vi "Project-SmartHome.vi"() -> ()   [LabVIEW 2013] (continued)
      }
      event "play": Value Change {
        n589 = event-data() -> ()  [unwired: 1 in, 6 out]
        n590 = local read "flag 7"() -> (w1128:u16)
        n591 = local read "channel"() -> (w1129:dbl)
        n592 = Equal?(x=w1128, y=w1129) -> (x = y?=w1135:bool)
        n593 = case shown="False" w1135 {
          tunnel: w1134 -> [w1139 w1156]
          tunnel: w1133 -> [w1144 w1159]
          tunnel: w1132 -> [w1143 w1160]
          tunnel: [w1142 w1158] -> w1131
          tunnel: [w1141 w1157] -> w1130
          tunnel: w1128 -> [w1137 _]
          frame False {
            n594 = To Double Precision Float(number=w1137) -> (double precision float=w1136:dbl)
            n595 = local read "flag 7"() -> (→"channel":u16)
            n596 = local read "URL"() -> (w1154:string)
            n597 = property class="IWMPPlayer4"(reference=w1139, "URL"=w1154) -> (reference out=w1153:refnum<k7>)  [unwired: 1 in, 1 out]
            n598 = property class="IWMPPlayer4"(reference=w1153) -> ("controls"=w1152:refnum<k7>)  [unwired: 1 in, 2 out]
            n599 = invoke class="IWMPControls" method="play"(reference=w1152) -> (reference out=w1151:refnum<k7>)  [unwired: 2 in, 2 out]
            n600 = Type Cast(x=8.0) -> (*(type *) &x=w1145:string)  [unwired: 1 in]
            n601 = TCP Write(connection ID=w1144, data in=w1145, error in (no error)=w1143) -> (connection ID out=w1147:refnum<k5>, error out=w1148:errorcluster)  [unwired: 1 in, 1 out]
            n602 = Close Reference(reference=w1151) -> ()  [unwired: 1 in, 1 out]
            n603 = Bundle(w1136, 1.0) -> (w1149:cluster{dbl, dbl})  [unwired: 1 in]
            n604 = Type Cast(x=w1149) -> (*(type *) &x=w1150:string)  [unwired: 1 in]
            n605 = TCP Write(connection ID=w1147, data in=w1150, error in (no error)=w1148) -> (connection ID out=w1142:refnum<k5>, error out=w1141:errorcluster)  [unwired: 1 in, 1 out]
          }
          frame True {
            n606 = property class="IWMPPlayer4"(reference=w1156) -> ("controls"=w1167:refnum<k7>)  [unwired: 1 in, 2 out]
            n607 = invoke class="IWMPControls" method="play"(reference=w1167) -> (reference out=w1168:refnum<k7>)  [unwired: 2 in, 2 out]
            n608 = Type Cast(x=7.0) -> (*(type *) &x=w1161:string)  [unwired: 1 in]
            n609 = TCP Write(connection ID=w1159, data in=w1161, error in (no error)=w1160) -> (connection ID out=w1163:refnum<k5>, error out=w1164:errorcluster)  [unwired: 1 in, 1 out]
            n610 = Bundle(2.0) -> (w1165:cluster{dbl})  [unwired: 1 in]
            n611 = Type Cast(x=w1165) -> (*(type *) &x=w1166:string)  [unwired: 1 in]
            n612 = Close Reference(reference=w1168) -> ()  [unwired: 1 in, 1 out]
            n613 = TCP Write(connection ID=w1163, data in=w1166, error in (no error)=w1164) -> (connection ID out=w1158:refnum<k5>, error out=w1157:errorcluster)  [unwired: 1 in, 1 out]
          }
        }
      }
      event "flag 7": Value Change {
        n614 = event-data() -> ()  [unwired: 1 in, 6 out]
        n615 = case shown="2" "flag 7" {
          frame 0, Default {
            "URL" <- "C:\\Users\\kiat\\Downloads\\asd.mp4" ("URL")
          }
          frame 1 {
            n616 = local write "URL"("C:\\Users\\kiat\\Downloads\\videoplayback.mp4" ("URL")) -> ()
          }
          frame 2 {
            n617 = local write "URL"("C:\\Users\\kiat\\Downloads\\wiggle.mp4" ("URL")) -> ()
          }
        }
      }
      event "backward": Value Change {
        n618 = event-data() -> ()  [unwired: 1 in, 6 out]
        n619 = Automation Open(Automation Refnum=w1185) -> (Automation Refnum=w1186:refnum<k7>)  [unwired: 3 in, 1 out]
        n620 = property class="IWMPPlayer4"(reference=w1186) -> ("controls"=w1187:refnum<k7>)  [unwired: 1 in, 2 out]
        n621 = invoke class="IWMPControls" method="fastReverse"(reference=w1187) -> (reference out=w1184:refnum<k7>)  [unwired: 2 in, 2 out]
        n622 = Type Cast(x=7.0) -> (*(type *) &x=w1178:string)  [unwired: 1 in]
        n623 = TCP Write(connection ID=w1176, data in=w1178, error in (no error)=w1175) -> (connection ID out=w1180:refnum<k5>, error out=w1181:errorcluster)  [unwired: 1 in, 1 out]
        n624 = Close Reference(reference=w1184) -> ()  [unwired: 1 in, 1 out]
        n625 = Bundle(5.0) -> (w1182:cluster{dbl})  [unwired: 1 in]
        n626 = Type Cast(x=w1182) -> (*(type *) &x=w1183:string)  [unwired: 1 in]
        n627 = TCP Write(connection ID=w1180, data in=w1183, error in (no error)=w1181) -> (connection ID out=w1174:refnum<k5>, error out=w1173:errorcluster)  [unwired: 1 in, 1 out]
      }
      event "foward": Value Change {
        n628 = event-data() -> ()  [unwired: 1 in, 6 out]
        n629 = Type Cast(x=7.0) -> (*(type *) &x=w1193:string)  [unwired: 1 in]
        n630 = TCP Write(connection ID=w1191, data in=w1193, error in (no error)=w1190) -> (connection ID out=w1195:refnum<k5>, error out=w1196:errorcluster)  [unwired: 1 in, 1 out]
        n631 = Bundle(6.0) -> (w1197:cluster{dbl})  [unwired: 1 in]
        n632 = Type Cast(x=w1197) -> (*(type *) &x=w1198:string)  [unwired: 1 in]
        n633 = TCP Write(connection ID=w1195, data in=w1198, error in (no error)=w1196) -> (connection ID out=w1189:refnum<k5>, error out=w1188:errorcluster)  [unwired: 1 in, 1 out]
        n634 = Automation Open(Automation Refnum=w1200) -> (Automation Refnum=w1201:refnum<k7>)  [unwired: 3 in, 1 out]
        n635 = property class="IWMPPlayer4"(reference=w1201) -> ("controls"=w1202:refnum<k7>)  [unwired: 1 in, 2 out]
        n636 = invoke class="IWMPControls" method="fastForward"(reference=w1202) -> (reference out=w1199:refnum<k7>)  [unwired: 2 in, 2 out]
        n637 = Close Reference(reference=w1199) -> ()  [unwired: 1 in, 1 out]
      }
      event "pause": Value Change {
        n638 = event-data() -> ()  [unwired: 1 in, 6 out]
        n639 = Automation Open(Automation Refnum=w1215) -> (Automation Refnum=w1214:refnum<k7>)  [unwired: 3 in, 1 out]
        n640 = property class="IWMPPlayer4"(reference=w1214) -> ("controls"=w1217:refnum<k7>)  [unwired: 1 in, 2 out]
        n641 = invoke class="IWMPControls" method="pause"(reference=w1217) -> (reference out=w1216:refnum<k7>)  [unwired: 2 in, 2 out]
        n642 = Type Cast(x=7.0) -> (*(type *) &x=w1208:string)  [unwired: 1 in]
        n643 = TCP Write(connection ID=w1203, data in=w1208, error in (no error)=w1204) -> (connection ID out=w1210:refnum<k5>, error out=w1211:errorcluster)  [unwired: 1 in, 1 out]
        n644 = Close Reference(reference=w1216) -> ()  [unwired: 1 in, 1 out]
        n645 = Bundle(3.0) -> (w1212:cluster{dbl})  [unwired: 1 in]
        n646 = Type Cast(x=w1212) -> (*(type *) &x=w1213:string)  [unwired: 1 in]
        n647 = TCP Write(connection ID=w1210, data in=w1213, error in (no error)=w1211) -> (connection ID out=w1206:refnum<k5>, error out=w1205:errorcluster)  [unwired: 1 in, 1 out]
      }
      event "add": Value Change {
        n648 = event-data() -> ()  [unwired: 1 in, 6 out]
        n649 = Read from Text File(file (use dialog)=w1219) -> (refnum out=w1220:refnum<file>, text=w1218:string)  [unwired: 3 in, 2 out]
        n650 = while {
          tunnel: w1218 -> [w1224]
          border: w1218 -> [_]
          stop <- w1222 stop-if-true
          n651 = feedback #1() -> (w1230:string)
          n652 = xnode "Match Regular Expression"("input string"=w1230, "regular expression"="\n") -> ("before match"=w1227:string, "after match"=w1231:string)  [unwired: 4 in, 3 out]
          n653 = feedback-in #1(w1231) -> ()
          n654 = Empty String/Path?(string/path=w1231) -> (empty?=w1221:bool)
          n655 = xnode "Match Regular Expression"("input string"=w1227, "regular expression"="-") -> ("before match"=w1228:string)  [unwired: 4 in, 4 out]
          n656 = local read "String"() -> (w1223:string)
          n657 = Equal?(x=w1223, y=w1228) -> (x = y?=w1225:bool)
          n658 = case shown="False" w1225 {
            tunnel: w1224 -> [w1233 _]
            tunnel: [w1232 w1261] -> w1222
            tunnel: w1221 -> [w1232 _]
            frame False {
              n659 = case shown="True" w1232 {
                tunnel: w1233 -> [_ w1238]
                frame False {
                }
                frame True {
                  n660 = case shown="1" "flag 8" {
                    tunnel: [w1259 w1260] -> w1242
                    tunnel: [w1259 w1260] -> w1246
                    frame 0, Default {
                      w1259 = "Admin"
                    }
                    frame 1 {
                      w1260 = "User"
                    }
                  }
                  n661 = Concatenate Strings("String", "-" ("string"), "String", ":" ("string"), w1242) -> (w1250:string)
                  n662 = local read "Numeric"() -> (w1249:dbl)
                  n663 = Open/Create/Replace File(file path (use dialog)=path "C:/Users/kiat/Desktop/password.txt" ("file (use dialog)")) -> (refnum out=w1236:refnum<file>)  [unwired: 5 in, 2 out]
                  n664 = local read "Table Control"() -> (w1247:string[][])
                  n665 = Build Array("String", "String", w1246) -> (w1243:string[])
                  n666 = case shown="0, Default" w1249 {
                    tunnel: [w1252 w1258] -> w1235
                    tunnel: w1238 -> [w1254 w1257]
                    tunnel: w1250 -> [w1253 w1255]
                    frame 0, Default {
                      n667 = Concatenate Strings(w1254, w1253) -> (w1252:string)
                      n668 = local write "Numeric"(0.0) -> ()
                    }
                    frame 1 {
                      n669 = Concatenate Strings(w1257, "\n", w1255) -> (w1258:string)
                    }
                  }
                  n670 = Write to Text File(file (use dialog)=w1236, text=w1235) -> (refnum out=w1237:refnum<file>)  [unwired: 2 in, 2 out]
                  n671 = Insert Into Array(array=w1247, new element=w1243) -> (w1248:string[][])  [unwired: 2 in]
                  n672 = local write "Table Control"(w1248) -> ()
                  n673 = Close File(refnum=w1237) -> ()  [unwired: 1 in, 2 out]
                }
              }
            }
            frame True {
              n674 = call "Display Message to User2"("Message"="Please choose another name") -> ("OK"=w1261:bool)  [unwired: 9 in, 1 out]
            }
          }
        }
        n675 = Close File(refnum=w1220) -> ()  [unwired: 1 in, 2 out]
      }
      event "edit": Value Change {
        n676 = event-data() -> ()  [unwired: 1 in, 6 out]
        n677 = property on="Table Control" class="Tbl (strict)"() -> ("Value"=w1486:string[][])  [unwired: 2 in, 2 out]
        n678 = local read "String"() -> (w1494:string)
        n679 = Read from Text File(file (use dialog)=w1493) -> (refnum out=w1507:refnum<file>, text=w1489:string, error out=w1513:errorcluster)  [unwired: 3 in, 1 out]
        n680 = Decimal String To Number(string=w1494) -> (number=w1487:i32)  [unwired: 2 in, 1 out]
        n681 = local read "Table Control"() -> (w1500:string[][])
        n682 = Array Size(array=w1486) -> (size(s)=w1496:i32[])
        n683 = local read "String"() -> (w1497:string)
        n684 = Add(x=1, y=w1487) -> (x+y=w1488:i32)
        n685 = Close File(refnum=w1507, error in=w1513) -> (path=w1504:path, error out=w1503:errorcluster)
        n686 = Index Array(array=w1496) -> (element=w1495:i32)  [unwired: 1 in]
        n687 = Decimal String To Number(string=w1497) -> (number=w1491:i32)  [unwired: 2 in, 1 out]
        n688 = Greater Or Equal?(x=w1488, y=w1495) -> (x >= y?=w1485:bool)
        n689 = case shown="True" w1485 {
          frame False {
          }
          frame True {
            n690 = local write "Table Control"(string[][] [] ("Table Control")) -> ()
            n691 = Read from Text File(file (use dialog)=path "C:/Users/kiat/Desktop/password.txt") -> (text=w1516:string)  [unwired: 3 in, 3 out]
            n692 = while {
              border: w1516 -> [_]
              stop <- w1526 stop-if-true
              n693 = feedback #2() -> (w1530:string)
              n694 = xnode "Match Regular Expression"("input string"=w1530, "regular expression"="\n") -> ("before match"=w1529:string, "after match"=w1528:string)  [unwired: 4 in, 3 out]
              n695 = feedback-in #2(w1528) -> ()
              n696 = xnode "Match Regular Expression"("input string"=w1529, "regular expression"="-") -> ("before match"=w1525:string, "after match"=w1524:string)  [unwired: 4 in, 3 out]
              n697 = Equal?(x=w1528, y="") -> (x = y?=w1526:bool)
              n698 = xnode "Match Regular Expression"("input string"=w1524, "regular expression"=":") -> ("before match"=w1521:string, "after match"=w1522:string)  [unwired: 4 in, 3 out]
              n699 = local read "Table Control"() -> (w1518:string[][])
              n700 = Build Array(w1525, w1521, w1522) -> (w1520:string[])
              n701 = Insert Into Array(array=w1518, new element=w1520) -> (w1519:string[][])  [unwired: 2 in]
              n702 = local write "Table Control"(w1519) -> ()
            }
          }
        }
        n703 = Index Array(array=w1500, index (row)=w1491, index (col)=0 ("index")) -> (element=w1502:string)
        n704 = local read "String"() -> (w1498:string)
        n705 = local read "Table Control"() -> (w1499:string[][])
        n706 = Open/Create/Replace File(file path (use dialog)=w1504, error in=w1503, operation (0:open)=T2."replace") -> (refnum out=w1511:refnum<file>, error out=w1510:errorcluster)  [unwired: 3 in, 1 out]
        n707 = Decimal String To Number(string=w1498) -> (number=w1492:i32)  [unwired: 2 in, 1 out]
        n708 = Index Array(array=w1499, index (row)=w1492, index (col)=1 ("index")) -> (element=w1508:string)
        n709 = while {
          tunnel: w1502 -> [w1889]
          tunnel: w1508 -> [w1888]
          border: "" -> [_]
          tunnel: [w1884] -> w1506
          border: w1489 -> [_]
          stop <- w1893 stop-if-true
          n710 = feedback #3() -> (w1891:string)
          n711 = xnode "Match Regular Expression"("input string"=w1891, "regular expression"="\n") -> ("before match"=w1887:string, "after match"=w1892:string)  [unwired: 4 in, 3 out]
          n712 = feedback-in #3(w1892) -> ()
          n713 = Empty String/Path?(string/path=w1892) -> (empty?=w1893:bool)
          n714 = xnode "Match Regular Expression"("input string"=w1887, "regular expression"="-") -> ("before match"=w1881:string, "after match"=w1883:string)  [unwired: 4 in, 3 out]
          n715 = xnode "Match Regular Expression"("input string"=w1883, "regular expression"=":") -> ("before match"=w1880:string)  [unwired: 4 in, 4 out]
          n716 = local read "flag 8"() -> (w1876:u16)
          n717 = case shown="1" w1876 {
            tunnel: ["Admin" "User"] -> w1875
            frame 0, Default {
            }
            frame 1 {
            }
          }
          n718 = Equal?(x=w1889, y=w1881) -> (x = y?=w1879:bool)
          n719 = Equal?(x=w1888, y=w1880) -> (x = y?=w1878:bool)
          n720 = And(x=w1879, y=w1878) -> (x .and. y?=w1877:bool)
          n721 = case shown="True" w1877 {
            tunnel: w1887 -> [w2009 w2018]
            tunnel: [w2008 w2017] -> w1886
            tunnel: w1875 -> [_ w2011]
            frame False {
              n722 = Concatenate Strings(w2009, "\n") -> (w2008:string)
            }
            frame True {
              n723 = local read "String"() -> (w2016:string)
              n724 = local read "String"() -> (w2014:string)
              n725 = Concatenate Strings(w2016, "-" ("string"), w2014, ":" ("string"), w2011) -> (w2012:string)
              n726 = Search and Replace String(input string=w2018, search string=w2018, replace string=w2012) -> (result string=w2017:string)  [unwired: 5 in, 3 out]
            }
          }
          n727 = feedback #4() -> (w1885:string)
          n728 = Concatenate Strings(w1885, w1886) -> (w1884:string)
          n729 = feedback-in #4(w1884) -> ()
        }
        n730 = Write to Text File(file (use dialog)=w1511, text=w1506, error in=w1510) -> (refnum out=w1505:refnum<file>)  [unwired: 1 in, 2 out]
        n731 = Close File(refnum=w1505) -> ()  [unwired: 1 in, 2 out]
      }
      event "delete": Value Change {
        n732 = event-data() -> ()  [unwired: 1 in, 6 out]
        n733 = property on="Table Control" class="Tbl (strict)"() -> ("Value"=w2245:string[][])  [unwired: 2 in, 2 out]
        n734 = Read from Text File(file (use dialog)=w2249) -> (refnum out=w2256:refnum<file>, text=w2261:string, error out=w2265:errorcluster)  [unwired: 3 in, 1 out]
        n735 = local read "String"() -> (w2251:string)
        n736 = Decimal String To Number(string=w2251) -> (number=w2250:i32)  [unwired: 2 in, 1 out]
        n737 = Array Size(array=w2245) -> (size(s)=w2254:i32[])
        n738 = local read "String"() -> (w2266:string)
        n739 = Index Array(array=w2254) -> (element=w2253:i32)  [unwired: 1 in]
        n740 = local read "Table Control"() -> (w2247:string[][])
        n741 = Close File(refnum=w2256, error in=w2265) -> (path=w2244:path, error out=w2243:errorcluster)
        n742 = Greater Or Equal?(x=w2250, y=w2253) -> (x >= y?=w2252:bool)
        n743 = Decimal String To Number(string=w2266) -> (number=w2268:i32)  [unwired: 2 in, 1 out]
        n744 = Index Array(array=w2247, index (row)=w2268, index (col)=0 ("index")) -> (element=w2242:string)
        n745 = case shown="False" w2252 {
          tunnel: w2250 -> [w2271 _]
          tunnel: w2245 -> [w2270 _]
          frame False {
            n746 = Delete From Array(array=w2270, length=1, index (row)=w2271) -> (array with subset deleted=w2269:string[][])  [unwired: 1 in, 1 out]
            n747 = property on="Table Control" class="Tbl (strict)"("Value"=w2269) -> ()  [unwired: 2 in, 2 out]
          }
          frame True {
          }
        }
        n748 = local read "String"() -> (w2260:string)
        n749 = local read "Table Control"() -> (w2246:string[][])
        n750 = Open/Create/Replace File(file path (use dialog)=w2244, error in=w2243, operation (0:open)=T2."replace") -> (refnum out=w2263:refnum<file>, error out=w2262:errorcluster)  [unwired: 3 in, 1 out]
        n751 = Decimal String To Number(string=w2260) -> (number=w2258:i32)  [unwired: 2 in, 1 out]
        n752 = Index Array(array=w2246, index (row)=w2258, index (col)=1 ("index")) -> (element=w2257:string)
        n753 = while {
          tunnel: w2261 -> [w2289]
          tunnel: w2242 -> [w2286]
          tunnel: w2257 -> [w2285]
          border: "" -> [_]
          tunnel: [w2278] -> w2255
          stop <- w2292 stop-if-true
          n754 = Wait Until Next ms Multiple(millisecond multiple=u32 2000) -> ()  [unwired: 1 out]
          n755 = feedback #5(w2289) -> (w2290:string)
          n756 = xnode "Match Regular Expression"("input string"=w2290, "regular expression"="\n") -> ("before match"=w2281:string, "after match"=w2291:string)  [unwired: 4 in, 3 out]
          n757 = feedback-in #5(w2291) -> ()
          n758 = Empty String/Path?(string/path=w2291) -> (empty?=w2292:bool)
          n759 = xnode "Match Regular Expression"("input string"=w2281, "regular expression"="-") -> ("before match"=w2287:string, "after match"=w2276:string)  [unwired: 4 in, 3 out]
          n760 = xnode "Match Regular Expression"("input string"=w2276, "regular expression"=":") -> ("before match"=w2274:string)  [unwired: 4 in, 4 out]
          n761 = Equal?(x=w2286, y=w2287) -> (x = y?=w2283:bool)
          n762 = Equal?(x=w2285, y=w2274) -> (x = y?=w2284:bool)
          n763 = And(x=w2283, y=w2284) -> (x .and. y?=w2282:bool)
          n764 = case shown="False" w2282 {
            tunnel: w2281 -> [w2406 w2410]
            tunnel: [w2405 w2408] -> w2280
            frame False {
              n765 = Concatenate Strings(w2406, "\n") -> (w2405:string)
            }
            frame True {
              n766 = Search and Replace String(input string=w2410, search string=w2410, replace string="" ("replace string (\"\")")) -> (result string=w2408:string)  [unwired: 5 in, 3 out]
            }
          }
          n767 = local write "Numeric"(0.0 ("Numeric")) -> ()
          n768 = feedback #6() -> (w2279:string)
          n769 = Concatenate Strings(w2279, w2280) -> (w2278:string)
          n770 = feedback-in #6(w2278) -> ()
        }
        n771 = Write to Text File(file (use dialog)=w2263, text=w2255, error in=w2262) -> (refnum out=w2248:refnum<file>)  [unwired: 1 in, 2 out]
        n772 = Close File(refnum=w2248) -> ()  [unwired: 1 in, 2 out]
      }
      event Value Change {
        n773 = event-data() -> ()  [unwired: 1 in, 6 out]
        n774 = property class="IWMPPlayer4"(reference=w2646) -> ("settings"=w2647:refnum<k7>)  [unwired: 1 in, 2 out]
        n775 = Type Cast(x=8.0) -> (*(type *) &x=w2639:string)  [unwired: 1 in]
        n776 = TCP Write(connection ID=w2638, data in=w2639, error in (no error)=w2637) -> (connection ID out=w2641:refnum<k5>, error out=w2642:errorcluster)  [unwired: 1 in, 1 out]
        n777 = Bundle("?", 2.0) -> (w2643:cluster{dbl, dbl})  [unwired: 1 in]
        n778 = Type Cast(x=w2643) -> (*(type *) &x=w2644:string)  [unwired: 1 in]
        n779 = TCP Write(connection ID=w2641, data in=w2644, error in (no error)=w2642) -> (connection ID out=w2636:refnum<k5>, error out=w2635:errorcluster)  [unwired: 1 in, 1 out]
        n780 = property class="IWMPSettings"(reference=w2647, "volume"="?") -> (reference out=w2645:refnum<k7>)  [unwired: 1 in, 1 out]
        n781 = Close Reference(reference=w2645) -> ()  [unwired: 1 in, 1 out]
      }
      event Value Change {
        n782 = event-data() -> ()  [unwired: 1 in, 6 out]
        n783 = property on="Tab Control" class="TabCtl (strict)"("Visible"=FALSE) -> ()  [unwired: 2 in, 2 out]
        n784 = property on="Tab Control 2" class="TabCtl (strict)"("Visible"=FALSE) -> ()  [unwired: 2 in, 2 out]
        n785 = property on="Tab Control 3" class="TabCtl (strict)"("Visible"=FALSE) -> ()  [unwired: 2 in, 2 out]
        n786 = property on="Tab Control 4" class="TabCtl (strict)"("Visible"=FALSE) -> ()  [unwired: 2 in, 2 out]
        n787 = property on="Tab Control 5" class="TabCtl (strict)"("Visible"=FALSE) -> ()  [unwired: 2 in, 2 out]
        n788 = property on="Tab Control 11" class="TabCtl (strict)"("Visible"=FALSE) -> ()  [unwired: 2 in, 2 out]
        n789 = property on="Tab Control 6" class="TabCtl (strict)"("Visible"=FALSE) -> ()  [unwired: 2 in, 2 out]
        n790 = property on="Tab Control 10" class="TabCtl (strict)"("Visible"=FALSE) -> ()  [unwired: 2 in, 2 out]
        n791 = property on="Tab Control 13" class="TabCtl (strict)"("Visible"=FALSE) -> ()  [unwired: 2 in, 2 out]
        n792 = property on="Tab Control 7" class="TabCtl (strict)"("Visible"=FALSE) -> ()  [unwired: 2 in, 2 out]
        n793 = property on="Tab Control 12" class="TabCtl (strict)"("Visible"=FALSE) -> ()  [unwired: 2 in, 2 out]
        n794 = property on="Tab Control 8" class="TabCtl (strict)"("Visible"=FALSE) -> ()  [unwired: 2 in, 2 out]
        n795 = property on="Tab Control 9" class="TabCtl (strict)"("Visible"=FALSE) -> ()  [unwired: 2 in, 2 out]
        n796 = property on="Tab Control 25" class="TabCtl (strict)"("Visible"=TRUE) -> ()  [unwired: 2 in, 2 out]
        n797 = property on="Tab Control 15" class="TabCtl (strict)"("Visible"=FALSE) -> ()  [unwired: 2 in, 2 out]
        n798 = property on="Tab Control 24" class="TabCtl (strict)"("Visible"=FALSE) -> ()  [unwired: 2 in, 2 out]
        n799 = property on="Tab Control 21" class="TabCtl (strict)"("Visible"=FALSE) -> ()  [unwired: 2 in, 2 out]
        n800 = property on="Tab Control 16" class="TabCtl (strict)"("Visible"=FALSE) -> ()  [unwired: 2 in, 2 out]
        n801 = property on="Tab Control 17" class="TabCtl (strict)"("Visible"=FALSE) -> ()  [unwired: 2 in, 2 out]
        n802 = property on="Tab Control 22" class="TabCtl (strict)"("Visible"=FALSE) -> ()  [unwired: 2 in, 2 out]
        n803 = property on="Tab Control 23" class="TabCtl (strict)"("Visible"=FALSE) -> ()  [unwired: 2 in, 2 out]
        n804 = property on="Tab Control 18" class="TabCtl (strict)"("Visible"=FALSE) -> ()  [unwired: 2 in, 2 out]
        n805 = property on="Tab Control 19" class="TabCtl (strict)"("Visible"=FALSE) -> ()  [unwired: 2 in, 2 out]
        n806 = property on="Tab Control 14" class="TabCtl (strict)"("Visible"=FALSE) -> ()  [unwired: 2 in, 2 out]
      }
      event "stop": Value Change {
        n807 = event-data() -> ()  [unwired: 1 in, 6 out]
        n808 = Type Cast(x=7.0) -> (*(type *) &x=w2677:string)  [unwired: 1 in]
        n809 = TCP Write(connection ID=w2675, data in=w2677, error in (no error)=w2674) -> (connection ID out=w2679:refnum<k5>, error out=w2680:errorcluster)  [unwired: 1 in, 1 out]
        n810 = Automation Open(Automation Refnum=w2684) -> (Automation Refnum=w2685:refnum<k7>)  [unwired: 3 in, 1 out]
        n811 = property class="IWMPPlayer4"(reference=w2685) -> ("controls"=w2686:refnum<k7>)  [unwired: 1 in, 2 out]
        n812 = invoke class="IWMPControls" method="stop"(reference=w2686) -> (reference out=w2683:refnum<k7>)  [unwired: 2 in, 2 out]
        n813 = Bundle(4.0) -> (w2681:cluster{dbl})  [unwired: 1 in]
        n814 = Type Cast(x=w2681) -> (*(type *) &x=w2682:string)  [unwired: 1 in]
        n815 = Close Reference(reference=w2683) -> ()  [unwired: 1 in, 1 out]
        n816 = TCP Write(connection ID=w2679, data in=w2682, error in (no error)=w2680) -> (connection ID out=w2673:refnum<k5>, error out=w2672:errorcluster)  [unwired: 1 in, 1 out]
      }
      event Value Change {
        # "Air conditional - Master room (set temperature)"
        n817 = event-data() -> ()  [unwired: 1 in, 6 out]
        n818 = Decimal String To Number(string="String") -> (number=w2693:i32)  [unwired: 2 in, 1 out]
        n819 = Type Cast(x=6.0) -> (*(type *) &x=w2694:string)  [unwired: 1 in]
        n820 = TCP Write(connection ID=w2689, data in=w2694, error in (no error)=w2690) -> (connection ID out=w2696:refnum<k5>, error out=w2697:errorcluster)  [unwired: 1 in, 1 out]
        n821 = Bundle("?", w2693, 2.0) -> (w2698:cluster{bool, i32, dbl})  [unwired: 1 in]
        n822 = Type Cast(x=w2698) -> (*(type *) &x=w2700:string)  [unwired: 1 in]
        n823 = TCP Write(connection ID=w2696, data in=w2700, error in (no error)=w2697) -> (connection ID out=w2688:refnum<k5>, error out=w2687:errorcluster)  [unwired: 1 in, 1 out]
      }
      event Value Change {
        # "Air conditional - Bed room (set temperature)"
        n824 = event-data() -> ()  [unwired: 1 in, 6 out]
        n825 = Decimal String To Number(string="String") -> (number=w2707:i32)  [unwired: 2 in, 1 out]
        n826 = Type Cast(x=6.0) -> (*(type *) &x=w2708:string)  [unwired: 1 in]
        n827 = TCP Write(connection ID=w2703, data in=w2708, error in (no error)=w2704) -> (connection ID out=w2710:refnum<k5>, error out=w2711:errorcluster)  [unwired: 1 in, 1 out]
        n828 = Bundle("?", w2707, 3.0) -> (w2712:cluster{bool, i32, dbl})  [unwired: 1 in]
        n829 = Type Cast(x=w2712) -> (*(type *) &x=w2714:string)  [unwired: 1 in]
        n830 = TCP Write(connection ID=w2710, data in=w2714, error in (no error)=w2711) -> (connection ID out=w2706:refnum<k5>, error out=w2705:errorcluster)  [unwired: 1 in, 1 out]
      }
      event Value Change {
        n831 = event-data() -> ()  [unwired: 1 in, 6 out]
        n832 = property on="Tab Control 6" class="TabCtl (strict)"("Visible"=FALSE) -> ()  [unwired: 2 in, 2 out]
        n833 = property on="Tab Control 21" class="TabCtl (strict)"("Visible"=FALSE) -> ()  [unwired: 2 in, 2 out]
        n834 = property on="Tab Control 10" class="TabCtl (strict)"("Visible"=FALSE) -> ()  [unwired: 2 in, 2 out]
        n835 = property on="Tab Control 8" class="TabCtl (strict)"("Visible"=FALSE) -> ()  [unwired: 2 in, 2 out]
        n836 = property on="Tab Control 9" class="TabCtl (strict)"("Visible"=FALSE) -> ()  [unwired: 2 in, 2 out]
        n837 = property on="Tab Control 5" class="TabCtl (strict)"("Visible"=FALSE) -> ()  [unwired: 2 in, 2 out]
        n838 = property on="Tab Control 12" class="TabCtl (strict)"("Visible"=FALSE) -> ()  [unwired: 2 in, 2 out]
        n839 = property on="Tab Control 7" class="TabCtl (strict)"("Visible"=FALSE) -> ()  [unwired: 2 in, 2 out]
        n840 = property on="Tab Control 22" class="TabCtl (strict)"("Visible"=FALSE) -> ()  [unwired: 2 in, 2 out]
        n841 = property on="Tab Control 11" class="TabCtl (strict)"("Visible"=FALSE) -> ()  [unwired: 2 in, 2 out]
        n842 = property on="Tab Control 4" class="TabCtl (strict)"("Visible"=FALSE) -> ()  [unwired: 2 in, 2 out]
        n843 = property on="Tab Control 3" class="TabCtl (strict)"("Visible"=FALSE) -> ()  [unwired: 2 in, 2 out]
        n844 = property on="Tab Control" class="TabCtl (strict)"("Visible"=FALSE) -> ()  [unwired: 2 in, 2 out]
        n845 = property on="Tab Control 2" class="TabCtl (strict)"("Visible"=FALSE) -> ()  [unwired: 2 in, 2 out]
        n846 = property on="Tab Control 19" class="TabCtl (strict)"("Visible"=FALSE) -> ()  [unwired: 2 in, 2 out]
        n847 = property on="Tab Control 14" class="TabCtl (strict)"("Visible"=FALSE) -> ()  [unwired: 2 in, 2 out]
        n848 = property on="Tab Control 16" class="TabCtl (strict)"("Visible"=FALSE) -> ()  [unwired: 2 in, 2 out]
        n849 = property on="Tab Control 13" class="TabCtl (strict)"("Visible"=FALSE) -> ()  [unwired: 2 in, 2 out]
        n850 = property on="Tab Control 15" class="TabCtl (strict)"("Visible"=TRUE) -> ()  [unwired: 2 in, 2 out]
        n851 = property on="Tab Control 24" class="TabCtl (strict)"("Visible"=FALSE) -> ()  [unwired: 2 in, 2 out]
        n852 = property on="Tab Control 18" class="TabCtl (strict)"("Visible"=FALSE) -> ()  [unwired: 2 in, 2 out]
        n853 = property on="Tab Control 17" class="TabCtl (strict)"("Visible"=FALSE) -> ()  [unwired: 2 in, 2 out]
      }
      event Value Change {
        n854 = event-data() -> ()  [unwired: 1 in, 6 out]
        n855 = Type Cast(x=4.0) -> (*(type *) &x=w2742:string)  [unwired: 1 in]
        n856 = TCP Write(connection ID=w2740, data in=w2742, error in (no error)=w2737) -> (connection ID out=w2739:refnum<k5>, error out=w2738:errorcluster)  [unwired: 1 in, 1 out]
        n857 = Bundle("?", 12.0) -> (w2747:cluster{bool, dbl})  [unwired: 1 in]
        n858 = Type Cast(x=w2747) -> (*(type *) &x=w2748:string)  [unwired: 1 in]
        n859 = TCP Write(connection ID=w2739, data in=w2748, error in (no error)=w2738) -> (connection ID out=w2745:refnum<k5>, error out=w2744:errorcluster)  [unwired: 1 in, 1 out]
      }
      event "OK Button 31": Value Change {
        n860 = event-data() -> ()  [unwired: 1 in, 6 out]
        n861 = Type Cast(x=4.0) -> (*(type *) &x=w2754:string)  [unwired: 1 in]
        n862 = TCP Write(connection ID=w2750, data in=w2754, error in (no error)=w2749) -> (connection ID out=w2751:refnum<k5>, error out=w2752:errorcluster)  [unwired: 1 in, 1 out]
        n863 = Bundle("OK Button 31"="OK Button 31", 13.0) -> (w2759:cluster{"OK Button 31":bool, dbl})  [unwired: 1 in]
        n864 = Type Cast(x=w2759) -> (*(type *) &x=w2760:string)  [unwired: 1 in]
        n865 = TCP Write(connection ID=w2751, data in=w2760, error in (no error)=w2752) -> (connection ID out=w2758:refnum<k5>, error out=w2757:errorcluster)  [unwired: 1 in, 1 out]
      }
      event "OK Button 32": Value Change {
        n866 = event-data() -> ()  [unwired: 1 in, 6 out]
        n867 = Type Cast(x=4.0) -> (*(type *) &x=w2769:string)  [unwired: 1 in]
        n868 = TCP Write(connection ID=w2762, data in=w2769, error in (no error)=w2763) -> (connection ID out=w2766:refnum<k5>, error out=w2767:errorcluster)  [unwired: 1 in, 1 out]
        n869 = Bundle("OK Button 32"="OK Button 32", 14.0) -> (w2771:cluster{"OK Button 32":bool, dbl})  [unwired: 1 in]
        n870 = Type Cast(x=w2771) -> (*(type *) &x=w2772:string)  [unwired: 1 in]
        n871 = TCP Write(connection ID=w2766, data in=w2772, error in (no error)=w2767) -> (connection ID out=w2765:refnum<k5>, error out=w2764:errorcluster)  [unwired: 1 in, 1 out]
      }
      event Value Change {
        n872 = event-data() -> ()  [unwired: 1 in, 6 out]
        n873 = Type Cast(x=4.0) -> (*(type *) &x=w2777:string)  [unwired: 1 in]
        n874 = TCP Write(connection ID=w2774, data in=w2777, error in (no error)=w2775) -> (connection ID out=w2773:refnum<k5>, error out=w2776:errorcluster)  [unwired: 1 in, 1 out]
        n875 = Bundle("?", 1.0) -> (w2783:cluster{bool, dbl})  [unwired: 1 in]
        n876 = Type Cast(x=w2783) -> (*(type *) &x=w2784:string)  [unwired: 1 in]
        n877 = TCP Write(connection ID=w2773, data in=w2784, error in (no error)=w2776) -> (connection ID out=w2781:refnum<k5>, error out=w2782:errorcluster)  [unwired: 1 in, 1 out]
      }
      event "OK Button 19": Value Change {
        n878 = event-data() -> ()  [unwired: 1 in, 6 out]
        n879 = Type Cast(x=4.0) -> (*(type *) &x=w2790:string)  [unwired: 1 in]
        n880 = TCP Write(connection ID=w2787, data in=w2790, error in (no error)=w2788) -> (connection ID out=w2786:refnum<k5>, error out=w2785:errorcluster)  [unwired: 1 in, 1 out]
        n881 = Bundle("OK Button 19"="OK Button 19", 2.0) -> (w2794:cluster{"OK Button 19":bool, dbl})  [unwired: 1 in]
        n882 = Type Cast(x=w2794) -> (*(type *) &x=w2796:string)  [unwired: 1 in]
        n883 = TCP Write(connection ID=w2786, data in=w2796, error in (no error)=w2785) -> (connection ID out=w2792:refnum<k5>, error out=w2793:errorcluster)  [unwired: 1 in, 1 out]
      }
      event "OK Button 20": Value Change {
        n884 = event-data() -> ()  [unwired: 1 in, 6 out]
        n885 = Type Cast(x=4.0) -> (*(type *) &x=w2802:string)  [unwired: 1 in]
        n886 = TCP Write(connection ID=w2799, data in=w2802, error in (no error)=w2800) -> (connection ID out=w2798:refnum<k5>, error out=w2797:errorcluster)  [unwired: 1 in, 1 out]
        n887 = Bundle("OK Button 20"="OK Button 20", 3.0) -> (w2803:cluster{"OK Button 20":bool, dbl})  [unwired: 1 in]
        n888 = Type Cast(x=w2803) -> (*(type *) &x=w2808:string)  [unwired: 1 in]
        n889 = TCP Write(connection ID=w2798, data in=w2808, error in (no error)=w2797) -> (connection ID out=w2806:refnum<k5>, error out=w2805:errorcluster)  [unwired: 1 in, 1 out]
      }
      event "OK Button 21": Value Change {
        n890 = event-data() -> ()  [unwired: 1 in, 6 out]
        n891 = Type Cast(x=4.0) -> (*(type *) &x=w2814:string)  [unwired: 1 in]
        n892 = TCP Write(connection ID=w2812, data in=w2814, error in (no error)=w2811) -> (connection ID out=w2809:refnum<k5>, error out=w2810:errorcluster)  [unwired: 1 in, 1 out]
        n893 = Bundle("OK Button 21"="OK Button 21", 4.0) -> (w2819:cluster{"OK Button 21":bool, dbl})  [unwired: 1 in]
        n894 = Type Cast(x=w2819) -> (*(type *) &x=w2820:string)  [unwired: 1 in]
        n895 = TCP Write(connection ID=w2809, data in=w2820, error in (no error)=w2810) -> (connection ID out=w2817:refnum<k5>, error out=w2816:errorcluster)  [unwired: 1 in, 1 out]
      }
      event "OK Button 22": Value Change {
        n896 = event-data() -> ()  [unwired: 1 in, 6 out]
        n897 = Type Cast(x=4.0) -> (*(type *) &x=w2826:string)  [unwired: 1 in]
        n898 = TCP Write(connection ID=w2823, data in=w2826, error in (no error)=w2822) -> (connection ID out=w2824:refnum<k5>, error out=w2821:errorcluster)  [unwired: 1 in, 1 out]
        n899 = Bundle("OK Button 22"="OK Button 22", 5.0) -> (w2831:cluster{"OK Button 22":bool, dbl})  [unwired: 1 in]
        n900 = Type Cast(x=w2831) -> (*(type *) &x=w2832:string)  [unwired: 1 in]
        n901 = TCP Write(connection ID=w2824, data in=w2832, error in (no error)=w2821) -> (connection ID out=w2829:refnum<k5>, error out=w2828:errorcluster)  [unwired: 1 in, 1 out]
      }
      event "OK Button 23": Value Change {
        n902 = event-data() -> ()  [unwired: 1 in, 6 out]
        n903 = Type Cast(x=4.0) -> (*(type *) &x=w2833:string)  [unwired: 1 in]
        n904 = TCP Write(connection ID=w2837, data in=w2833, error in (no error)=w2836) -> (connection ID out=w2834:refnum<k5>, error out=w2835:errorcluster)  [unwired: 1 in, 1 out]
        n905 = Bundle("OK Button 23"="OK Button 23", 6.0) -> (w2843:cluster{"OK Button 23":bool, dbl})  [unwired: 1 in]
        n906 = Type Cast(x=w2843) -> (*(type *) &x=w2844:string)  [unwired: 1 in]
        n907 = TCP Write(connection ID=w2834, data in=w2844, error in (no error)=w2835) -> (connection ID out=w2841:refnum<k5>, error out=w2840:errorcluster)  [unwired: 1 in, 1 out]
      }
      event "OK Button 24": Value Change {
        n908 = event-data() -> ()  [unwired: 1 in, 6 out]
        n909 = Type Cast(x=4.0) -> (*(type *) &x=w2845:string)  [unwired: 1 in]
        n910 = TCP Write(connection ID=w2850, data in=w2845, error in (no error)=w2849) -> (connection ID out=w2851:refnum<k5>, error out=w2852:errorcluster)  [unwired: 1 in, 1 out]
        n911 = Bundle("OK Button 24"="OK Button 24", 7.0) -> (w2855:cluster{"OK Button 24":bool, dbl})  [unwired: 1 in]
        n912 = Type Cast(x=w2855) -> (*(type *) &x=w2856:string)  [unwired: 1 in]
        n913 = TCP Write(connection ID=w2851, data in=w2856, error in (no error)=w2852) -> (connection ID out=w2848:refnum<k5>, error out=w2847:errorcluster)  [unwired: 1 in, 1 out]
      }
      event Value Change {
        n914 = event-data() -> ()  [unwired: 1 in, 6 out]
        n915 = Type Cast(x=4.0) -> (*(type *) &x=w2862:string)  [unwired: 1 in]
        n916 = TCP Write(connection ID=w2858, data in=w2862, error in (no error)=w2857) -> (connection ID out=w2859:refnum<k5>, error out=w2860:errorcluster)  [unwired: 1 in, 1 out]
        n917 = Bundle("?", 8.0) -> (w2867:cluster{bool, dbl})  [unwired: 1 in]
        n918 = Type Cast(x=w2867) -> (*(type *) &x=w2868:string)  [unwired: 1 in]
        n919 = TCP Write(connection ID=w2859, data in=w2868, error in (no error)=w2860) -> (connection ID out=w2864:refnum<k5>, error out=w2863:errorcluster)  [unwired: 1 in, 1 out]
      }
      event "OK Button 25": Value Change {
        n920 = event-data() -> ()  [unwired: 1 in, 6 out]
        n921 = Type Cast(x=4.0) -> (*(type *) &x=w2874:string)  [unwired: 1 in]
        n922 = TCP Write(connection ID=w2869, data in=w2874, error in (no error)=w2872) -> (connection ID out=w2870:refnum<k5>, error out=w2871:errorcluster)  [unwired: 1 in, 1 out]
        n923 = Bundle("OK Button 25"="OK Button 25", 9.0) -> (w2879:cluster{"OK Button 25":bool, dbl})  [unwired: 1 in]
        n924 = Type Cast(x=w2879) -> (*(type *) &x=w2880:string)  [unwired: 1 in]
        n925 = TCP Write(connection ID=w2870, data in=w2880, error in (no error)=w2871) -> (connection ID out=w2877:refnum<k5>, error out=w2876:errorcluster)  [unwired: 1 in, 1 out]
      }
      event "OK Button 26": Value Change {
        n926 = event-data() -> ()  [unwired: 1 in, 6 out]
        n927 = Type Cast(x=4.0) -> (*(type *) &x=w2886:string)  [unwired: 1 in]
        n928 = TCP Write(connection ID=w2884, data in=w2886, error in (no error)=w2883) -> (connection ID out=w2882:refnum<k5>, error out=w2881:errorcluster)  [unwired: 1 in, 1 out]
        n929 = Bundle("OK Button 26"="OK Button 26", 10.0) -> (w2891:cluster{"OK Button 26":bool, dbl})  [unwired: 1 in]
        n930 = Type Cast(x=w2891) -> (*(type *) &x=w2892:string)  [unwired: 1 in]
        n931 = TCP Write(connection ID=w2882, data in=w2892, error in (no error)=w2881) -> (connection ID out=w2889:refnum<k5>, error out=w2888:errorcluster)  [unwired: 1 in, 1 out]
      }
      event "OK Button 27": Value Change {
        n932 = event-data() -> ()  [unwired: 1 in, 6 out]
        n933 = Type Cast(x=4.0) -> (*(type *) &x=w2898:string)  [unwired: 1 in]
        n934 = TCP Write(connection ID=w2896, data in=w2898, error in (no error)=w2893) -> (connection ID out=w2895:refnum<k5>, error out=w2894:errorcluster)  [unwired: 1 in, 1 out]
        n935 = Bundle("OK Button 27"="OK Button 27", 11.0) -> (w2903:cluster{"OK Button 27":bool, dbl})  [unwired: 1 in]
        n936 = Type Cast(x=w2903) -> (*(type *) &x=w2904:string)  [unwired: 1 in]
        n937 = TCP Write(connection ID=w2895, data in=w2904, error in (no error)=w2894) -> (connection ID out=w2901:refnum<k5>, error out=w2900:errorcluster)  [unwired: 1 in, 1 out]
      }
      event Value Change {
        (unwired) FALSE ("Visible")
        n938 = event-data() -> ()  [unwired: 1 in, 6 out]
        n939 = property on="Tab Control 8" class="TabCtl (strict)"("Visible"=FALSE) -> ()  [unwired: 2 in, 2 out]
        n940 = property on="Tab Control 6" class="TabCtl (strict)"("Visible"=FALSE) -> ()  [unwired: 2 in, 2 out]
        n941 = property on="Tab Control 9" class="TabCtl (strict)"("Visible"=FALSE) -> ()  [unwired: 2 in, 2 out]
        n942 = property on="Tab Control 19" class="TabCtl (strict)"("Visible"=FALSE) -> ()  [unwired: 2 in, 2 out]
        n943 = property on="Tab Control 22" class="TabCtl (strict)"("Visible"=FALSE) -> ()  [unwired: 2 in, 2 out]
        n944 = property on="Tab Control 12" class="TabCtl (strict)"("Visible"=FALSE) -> ()  [unwired: 2 in, 2 out]
        n945 = property on="Tab Control 5" class="TabCtl (strict)"("Visible"=TRUE) -> ()  [unwired: 2 in, 2 out]
        n946 = property on="Tab Control 4" class="TabCtl (strict)"("Visible"=FALSE) -> ()  [unwired: 2 in, 2 out]
        n947 = property on="Tab Control 3" class="TabCtl (strict)"("Visible"=FALSE) -> ()  [unwired: 2 in, 2 out]
        n948 = property on="Tab Control" class="TabCtl (strict)"("Visible"=FALSE) -> ()  [unwired: 2 in, 2 out]
        n949 = property on="Tab Control 2" class="TabCtl (strict)"("Visible"=FALSE) -> ()  [unwired: 2 in, 2 out]
        n950 = property on="Tab Control 21" class="TabCtl (strict)"("Visible"=FALSE) -> ()  [unwired: 2 in, 2 out]
        n951 = property on="Tab Control 10" class="TabCtl (strict)"("Visible"=FALSE) -> ()  [unwired: 2 in, 2 out]
        n952 = property on="Tab Control 7" class="TabCtl (strict)"("Visible"=FALSE) -> ()  [unwired: 2 in, 2 out]
        n953 = property on="Tab Control 11" class="TabCtl (strict)"("Visible"=FALSE) -> ()  [unwired: 2 in, 2 out]
        n954 = property on="Tab Control 16" class="TabCtl (strict)"("Visible"=FALSE) -> ()  [unwired: 2 in, 2 out]
        n955 = property on="Tab Control 14" class="TabCtl (strict)"("Visible"=FALSE) -> ()  [unwired: 2 in, 2 out]
        n956 = property on="Tab Control 13" class="TabCtl (strict)"("Visible"=FALSE) -> ()  [unwired: 2 in, 2 out]
        n957 = property on="Tab Control 15" class="TabCtl (strict)"("Visible"=FALSE) -> ()  [unwired: 2 in, 2 out]
        n958 = property on="Tab Control 18" class="TabCtl (strict)"("Visible"=FALSE) -> ()  [unwired: 2 in, 2 out]
        n959 = property on="Tab Control 17" class="TabCtl (strict)"("Visible"=FALSE) -> ()  [unwired: 2 in, 2 out]
        n960 = property on="Tab Control 24" class="TabCtl (strict)"("Visible"=FALSE) -> ()  [unwired: 2 in, 2 out]
      }
      event Value Change {
        n961 = event-data() -> ()  [unwired: 1 in, 6 out]
        n962 = Type Cast(x=0.0) -> ()  [unwired: 1 in, 1 out]
        n963 = TCP Write(connection ID=w2927, error in (no error)=w2928) -> (connection ID out=w2930:refnum<k5>, error out=w2929:errorcluster)  [unwired: 2 in, 1 out]
        n964 = Bundle("?", 3.0) -> (w2936:cluster{bool, dbl})  [unwired: 1 in]
        n965 = Type Cast(x=w2936) -> (*(type *) &x=w2937:string)  [unwired: 1 in]
        n966 = TCP Write(connection ID=w2930, data in=w2937, error in (no error)=w2929) -> (connection ID out=w2933:refnum<k5>, error out=w2932:errorcluster)  [unwired: 1 in, 1 out]
      }
      event "OK Button 11": Value Change {
        n967 = event-data() -> ()  [unwired: 1 in, 6 out]
        n968 = Type Cast(x=0.0) -> (*(type *) &x=w2943:string)  [unwired: 1 in]
        n969 = TCP Write(connection ID=w2940, data in=w2943, error in (no error)=w2941) -> (connection ID out=w2939:refnum<k5>, error out=w2938:errorcluster)  [unwired: 1 in, 1 out]
        n970 = Bundle("OK Button 11"="OK Button 11", 4.0) -> (w2948:cluster{"OK Button 11":bool, dbl})  [unwired: 1 in]
        n971 = Type Cast(x=w2948) -> (*(type *) &x=w2949:string)  [unwired: 1 in]
        n972 = TCP Write(connection ID=w2939, data in=w2949, error in (no error)=w2938) -> (connection ID out=w2945:refnum<k5>, error out=w2944:errorcluster)  [unwired: 1 in, 1 out]
      }
      event "OK Button 12": Value Change {
        n973 = event-data() -> ()  [unwired: 1 in, 6 out]
        n974 = Type Cast(x=0.0) -> (*(type *) &x=w2955:string)  [unwired: 1 in]
        n975 = TCP Write(connection ID=w2953, data in=w2955, error in (no error)=w2950) -> (connection ID out=w2952:refnum<k5>, error out=w2951:errorcluster)  [unwired: 1 in, 1 out]
        n976 = Bundle("OK Button 12"="OK Button 12", 8.0) -> (w2960:cluster{"OK Button 12":bool, dbl})  [unwired: 1 in]
        n977 = Type Cast(x=w2960) -> (*(type *) &x=w2961:string)  [unwired: 1 in]
        n978 = TCP Write(connection ID=w2952, data in=w2961, error in (no error)=w2951) -> (connection ID out=w2957:refnum<k5>, error out=w2958:errorcluster)  [unwired: 1 in, 1 out]
      }
      event "OK Button 13": Value Change {
        n979 = event-data() -> ()  [unwired: 1 in, 6 out]
        n980 = Type Cast(x=0.0) -> (*(type *) &x=w2967:string)  [unwired: 1 in]
        n981 = TCP Write(connection ID=w2965, data in=w2967, error in (no error)=w2962) -> (connection ID out=w2964:refnum<k5>, error out=w2963:errorcluster)  [unwired: 1 in, 1 out]
        n982 = Bundle("OK Button 13"="OK Button 13", 9.0) -> (w2972:cluster{"OK Button 13":bool, dbl})  [unwired: 1 in]
        n983 = Type Cast(x=w2972) -> (*(type *) &x=w2973:string)  [unwired: 1 in]
        n984 = TCP Write(connection ID=w2964, data in=w2973, error in (no error)=w2963) -> (connection ID out=w2969:refnum<k5>, error out=w2970:errorcluster)  [unwired: 1 in, 1 out]
      }
      event "OK Button 14": Value Change {
        n985 = event-data() -> ()  [unwired: 1 in, 6 out]
        n986 = Type Cast(x=0.0) -> ()  [unwired: 1 in, 1 out]
        n987 = TCP Write(connection ID=w2975, error in (no error)=w2974) -> (connection ID out=w2976:refnum<k5>, error out=w2977:errorcluster)  [unwired: 2 in, 1 out]
        n988 = Bundle("OK Button 14"="OK Button 14", 19.0) -> (w2983:cluster{"OK Button 14":bool, dbl})  [unwired: 1 in]
        n989 = Type Cast(x=w2983) -> (*(type *) &x=w2984:string)  [unwired: 1 in]
        n990 = TCP Write(connection ID=w2976, data in=w2984, error in (no error)=w2977) -> (connection ID out=w2981:refnum<k5>, error out=w2982:errorcluster)  [unwired: 1 in, 1 out]
      }
      event Value Change {
        n991 = event-data() -> ()  [unwired: 1 in, 6 out]
        n992 = Type Cast(x=0.0) -> (*(type *) &x=w2990:string)  [unwired: 1 in]
        n993 = TCP Write(connection ID=w2986, data in=w2990, error in (no error)=w2985) -> (connection ID out=w2987:refnum<k5>, error out=w2988:errorcluster)  [unwired: 1 in, 1 out]